vi "Velociprobe_Nanopositioner_Control_RT 3.vi"() -> ()   [LabVIEW 2015] (continued)
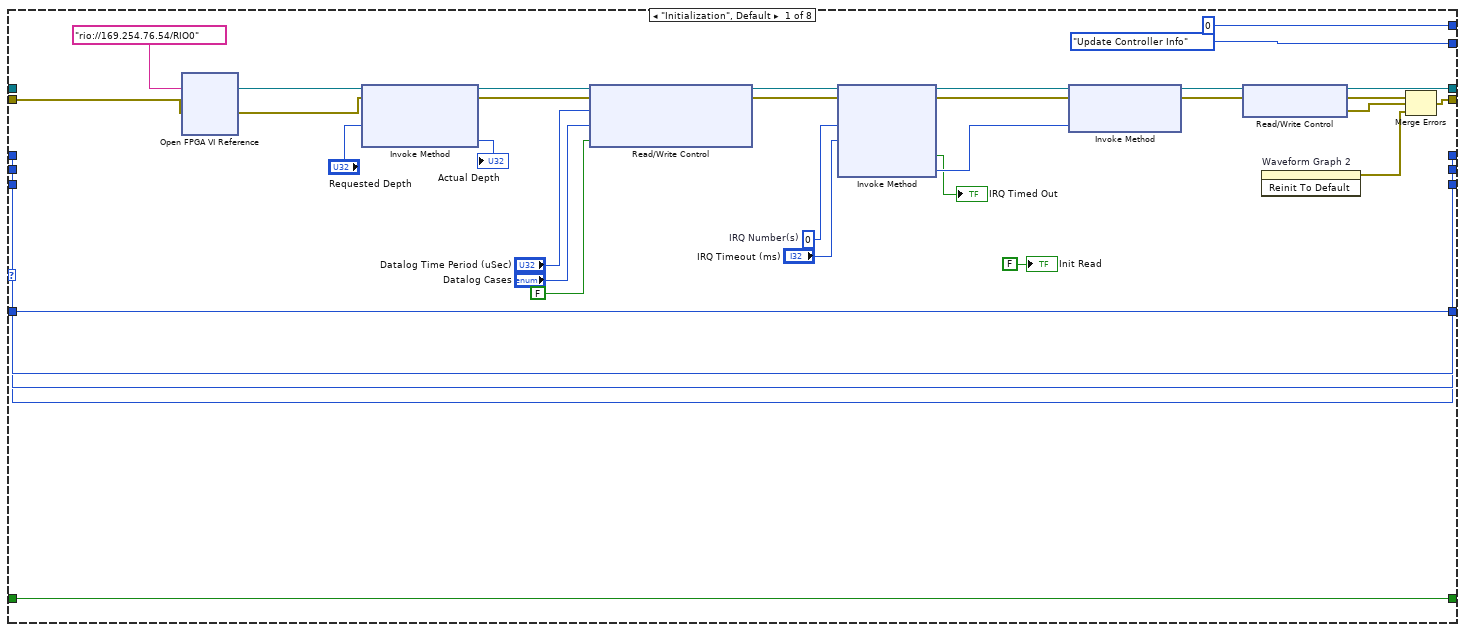
[diagram p2: hidden frame]
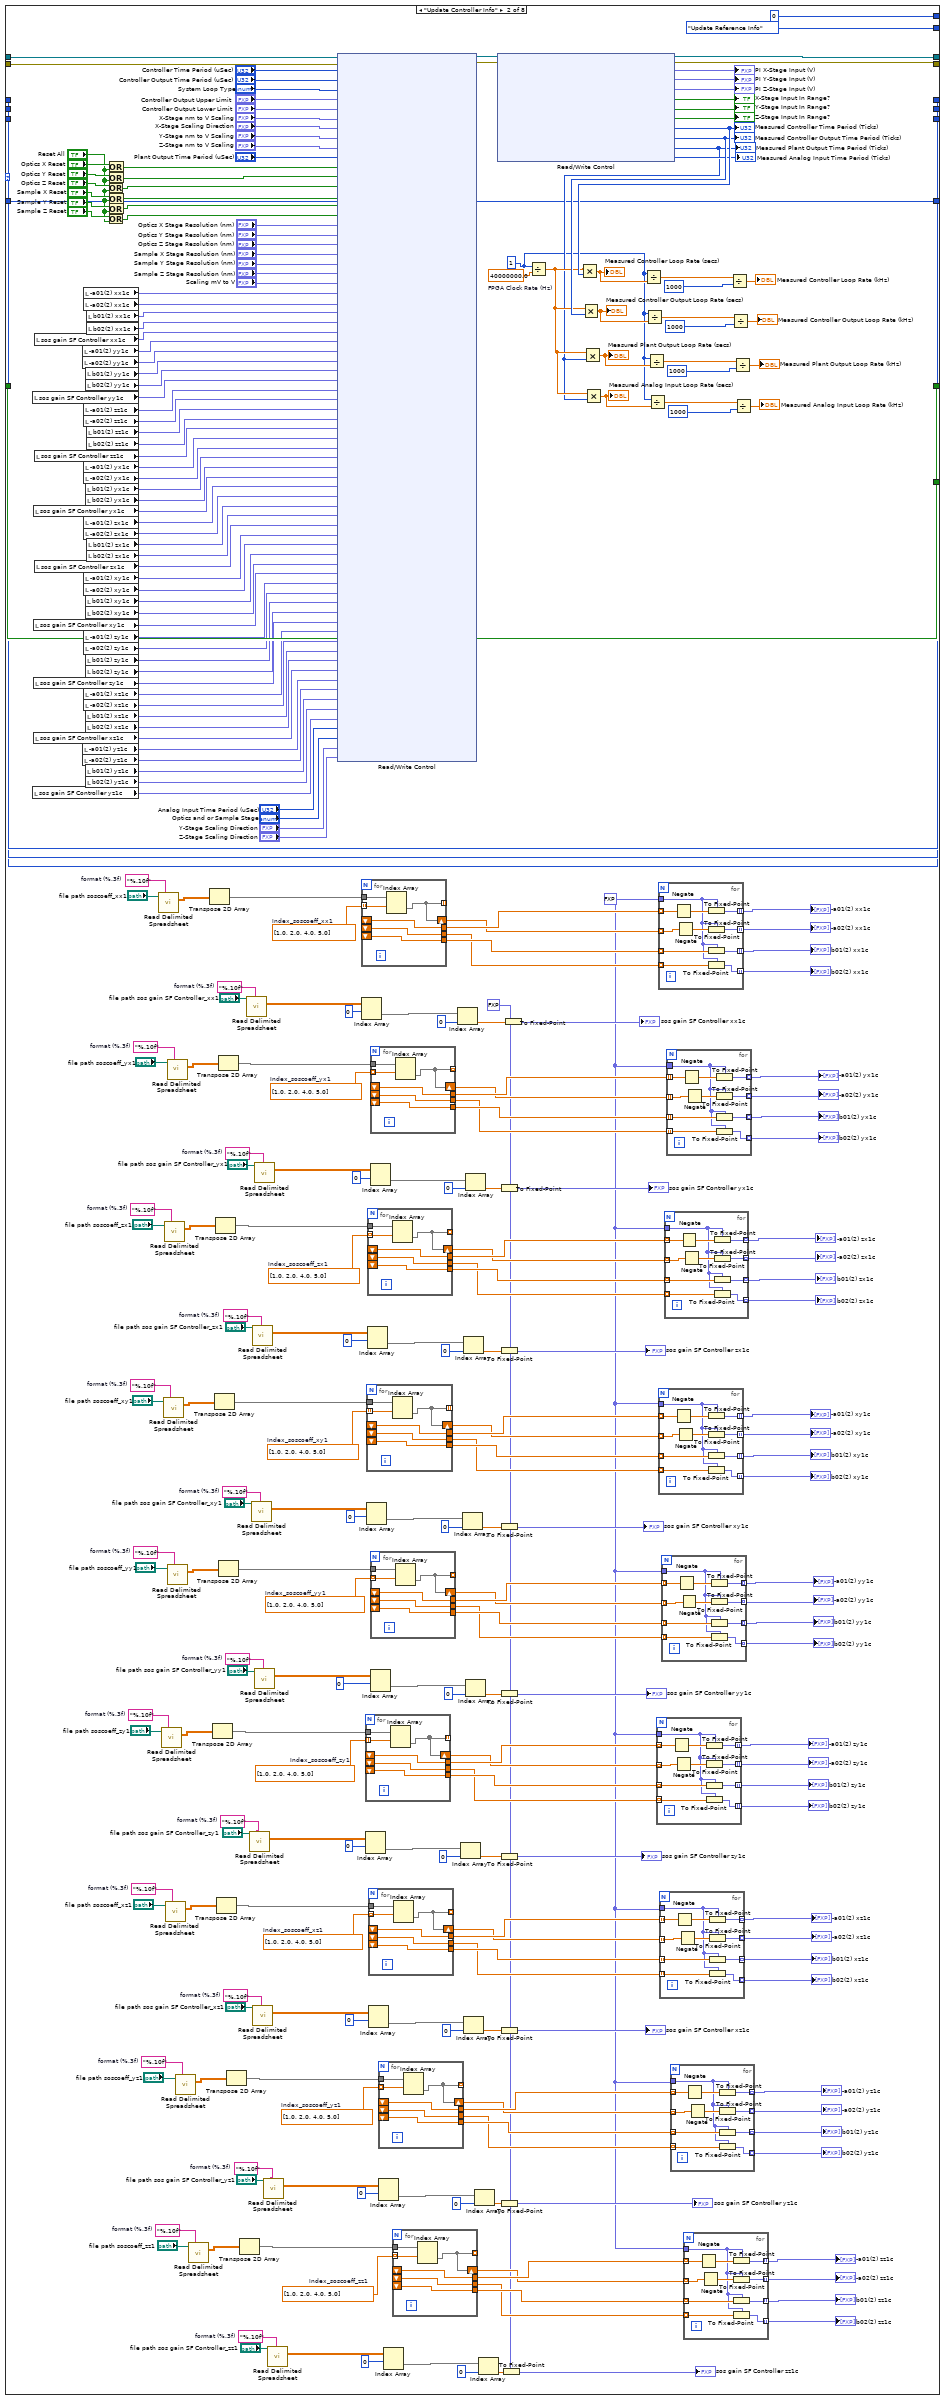
[diagram p3: hidden frame]
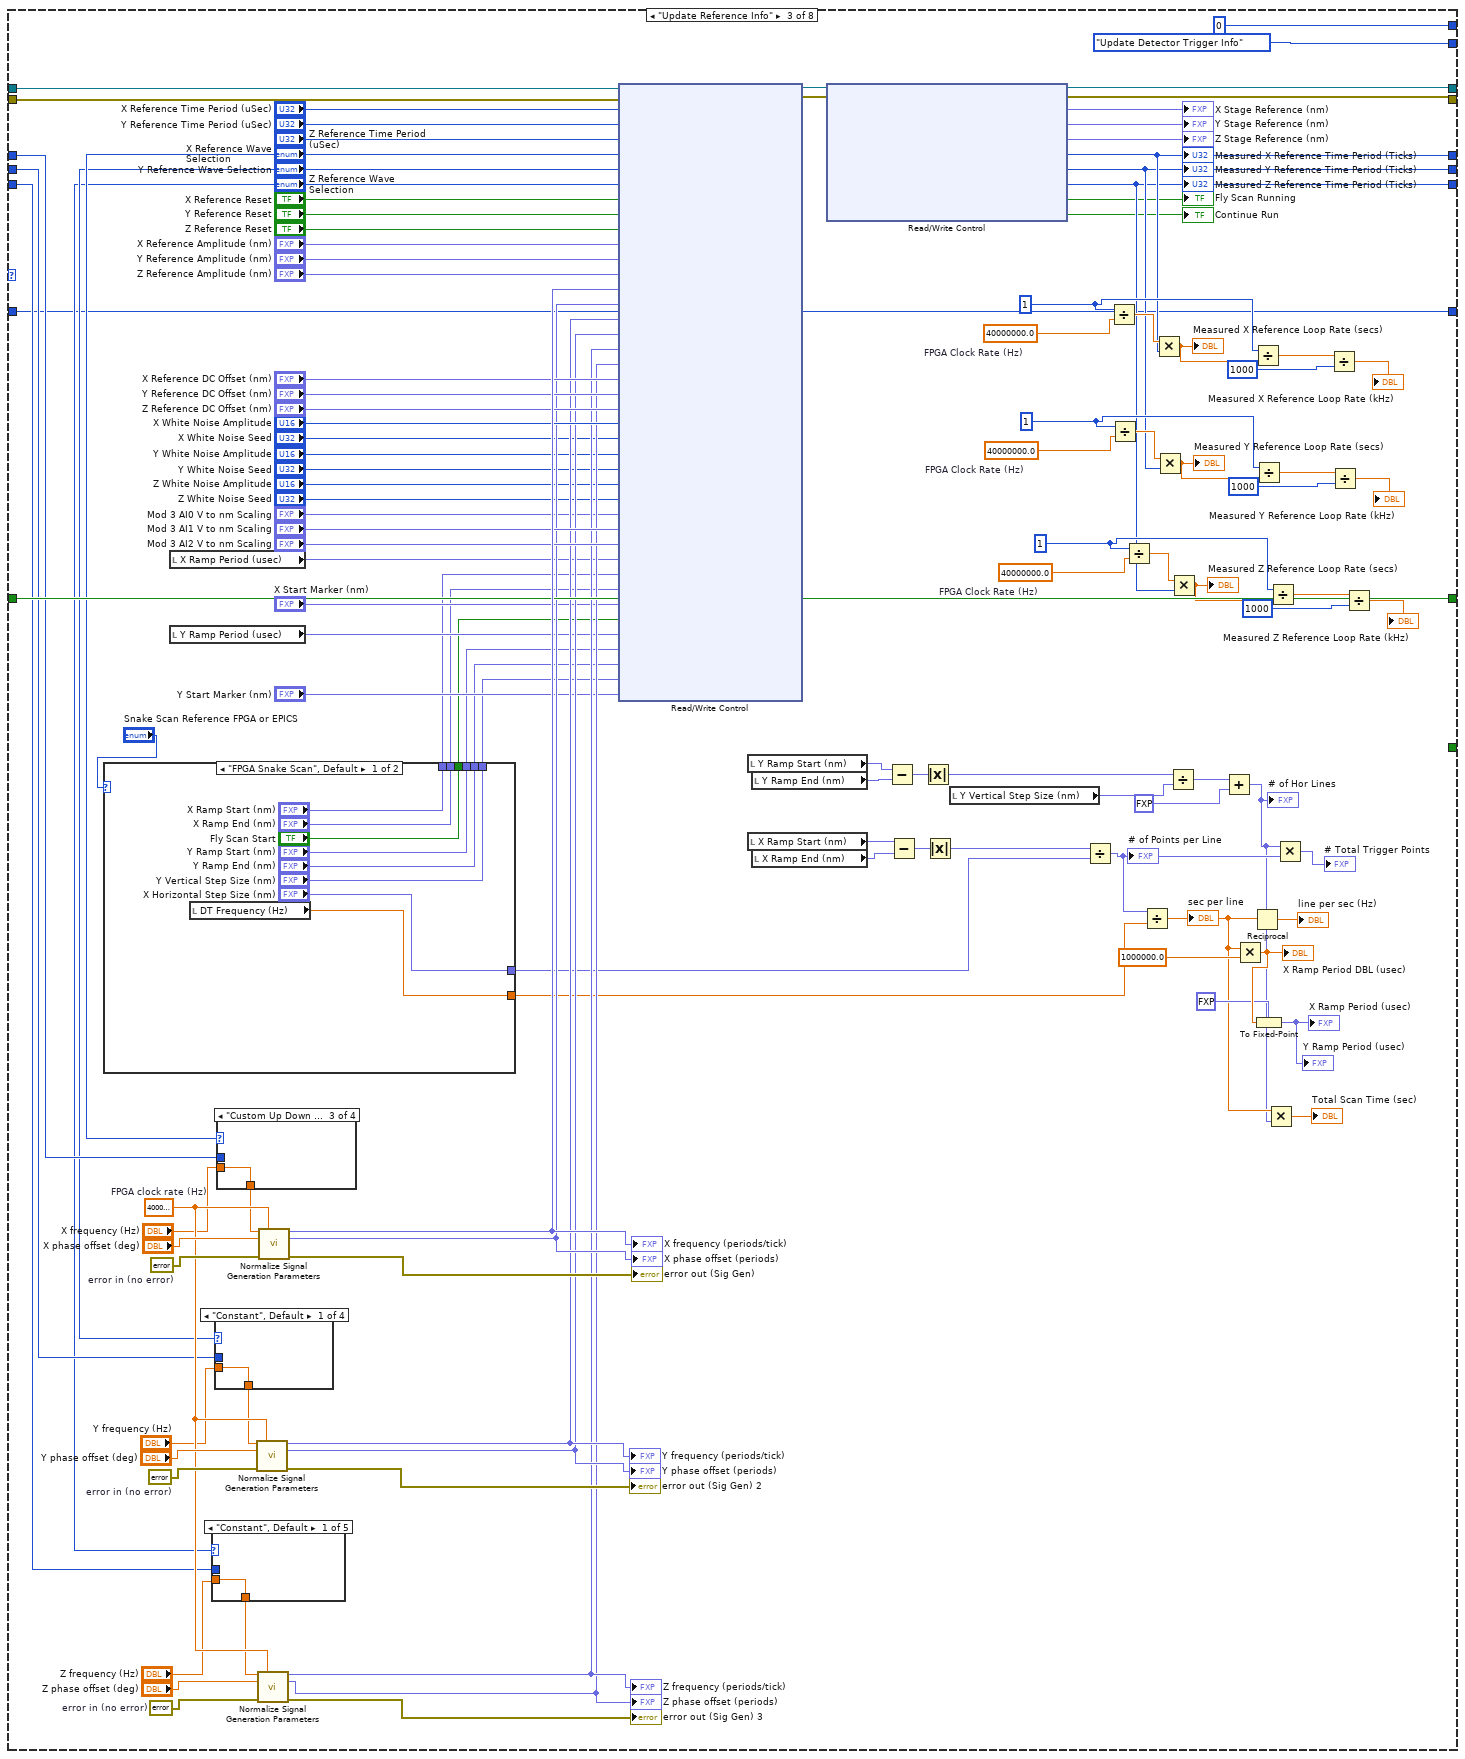
[diagram p4: hidden frame]
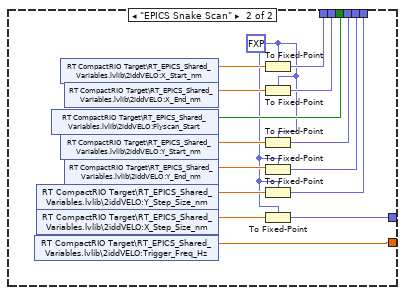
[diagram p5: hidden frame]
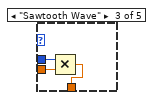
[diagram p7: hidden frame]
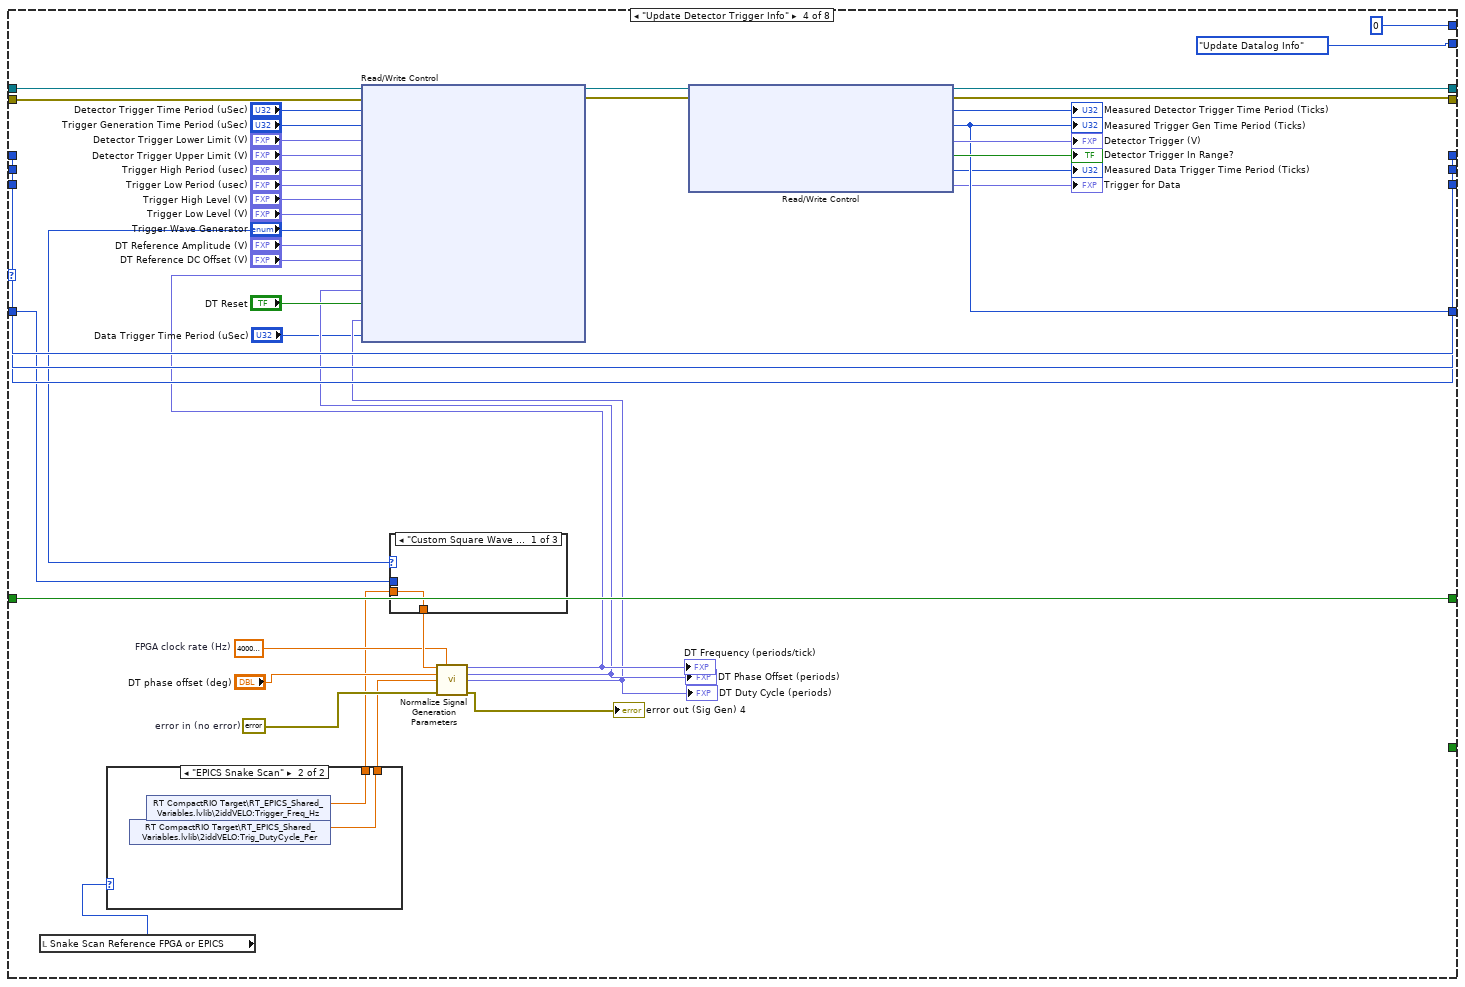
[diagram p16: hidden frame]
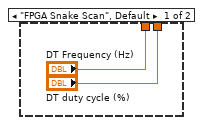
[diagram p17: hidden frame]
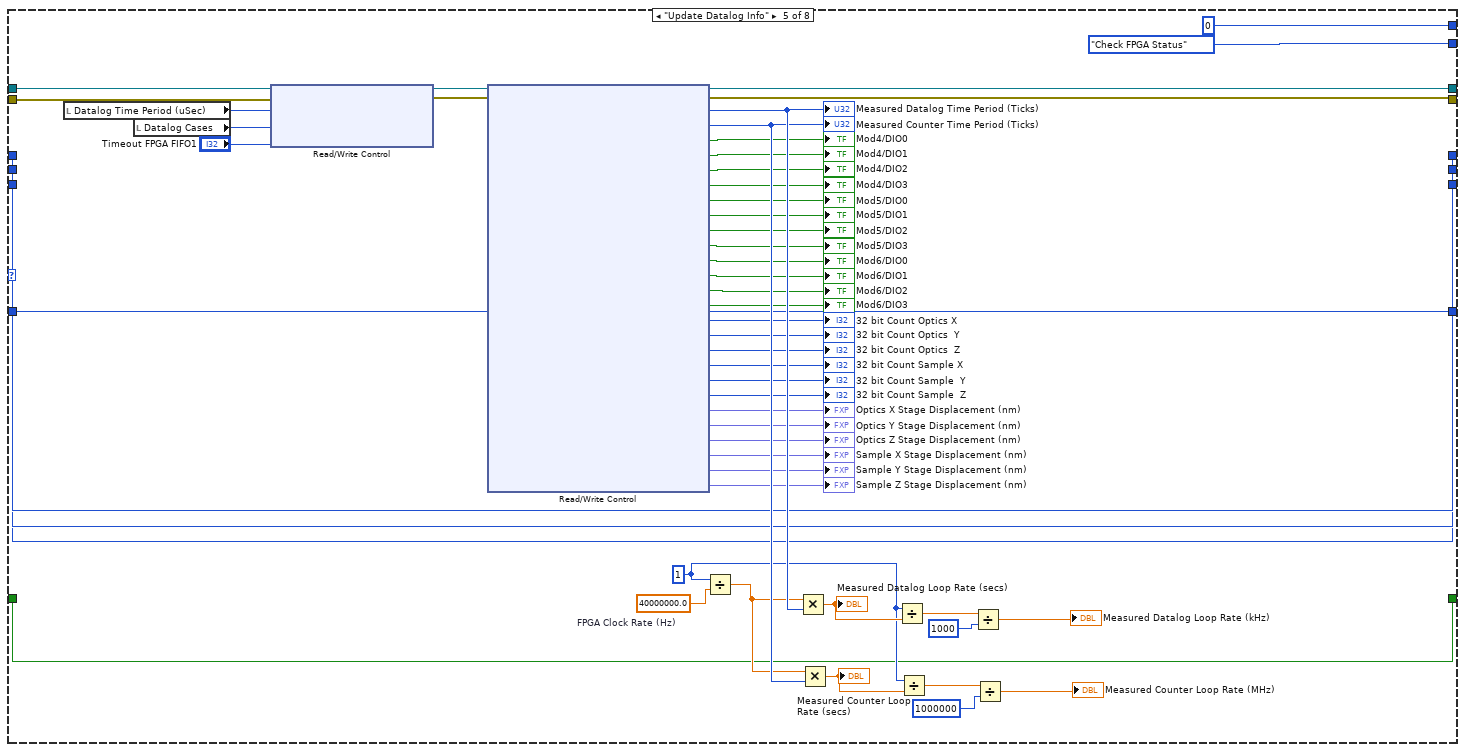
[diagram p20: hidden frame]
            n221 = shared-variable "RT CompactRIO Target\\RT_EPICS_Shared_Variables.lvlib\\2iddVELO:Flyscan_Start"() -> (w667:bool)  [unwired: 1 in, 1 out]
            n222 = shared-variable "RT CompactRIO Target\\RT_EPICS_Shared_Variables.lvlib\\2iddVELO:X_Start_nm"() -> (w675:dbl)  [unwired: 1 in, 1 out]
            n223 = shared-variable "RT CompactRIO Target\\RT_EPICS_Shared_Variables.lvlib\\2iddVELO:Y_Start_nm"() -> (w673:dbl)  [unwired: 1 in, 1 out]
            n224 = shared-variable "RT CompactRIO Target\\RT_EPICS_Shared_Variables.lvlib\\2iddVELO:X_End_nm"() -> (w674:dbl)  [unwired: 1 in, 1 out]
            n225 = shared-variable "RT CompactRIO Target\\RT_EPICS_Shared_Variables.lvlib\\2iddVELO:Y_End_nm"() -> (w672:dbl)  [unwired: 1 in, 1 out]
            n226 = To Fixed-Point(fixed-point type=w662, number=w675) -> (fixed-point=w669:fxp<+/-,16,16>)
            n227 = To Fixed-Point(fixed-point type=w662, number=w674) -> (fixed-point=w668:fxp<+/-,16,16>)
            n228 = To Fixed-Point(fixed-point type=w662, number=w673) -> (fixed-point=w666:fxp<+/-,16,16>)
            n229 = To Fixed-Point(fixed-point type=w662, number=w672) -> (fixed-point=w665:fxp<+/-,16,16>)
            n230 = To Fixed-Point(fixed-point type=w662, number=w671) -> (fixed-point=w664:fxp<+/-,16,16>)
            n231 = To Fixed-Point(fixed-point type=w662, number=w670) -> (fixed-point=w663:fxp<+/-,16,16>)
          }
        }
        n232 = local read "X Ramp Period (usec)"() -> (w551:fxp<+,24,24>)
        n233 = local read "Y Ramp Period (usec)"() -> (w552:fxp<+,24,24>)
        n234 = case shown="\"Constant\", Default" "Z Reference Wave Selection" {
          tunnel: "Z frequency (Hz)" -> [w676 w677 w679 w681 w682]
          tunnel: [w676 w677 w678 w681 w682] -> w577
          tunnel: w576 -> [_ _ w680 _ _]
          frame "Constant", Default {
          }
          frame "Sine Wave" {
          }
          frame "Sawtooth Wave" {
            n235 = Multiply(x=w680, y=w679) -> (x*y=w678:dbl)
          }
          frame "Square Wave" {
          }
          frame "Filtered White Noise" {
          }
        }
        n236 = case shown="\"Constant\", Default" "Y Reference Wave Selection" {
          tunnel: "Y frequency (Hz)" -> [w683 w684 w685 w686]
          tunnel: [w683 w684 w685 w686] -> w582
          tunnel: w579 -> [_ _ _ _]
          frame "Constant", Default {
          }
          frame "Sine Wave" {
          }
          frame "Custom Ramp Wave" {
          }
          frame "Filtered White Noise" {
          }
        }
        n237 = case shown="\"Custom Up Down Ramp\"" "X Reference Wave Selection" {
          tunnel: "X frequency (Hz)" -> [w687 w688 w689 w690]
          tunnel: [w687 w688 w689 w690] -> w586
          tunnel: w584 -> [_ _ _ _]
          frame "Constant", Default {
          }
          frame "Sine Wave" {
          }
          frame "Custom Up Down Ramp" {
          }
          frame "Filtered White Noise" {
          }
        }
        n238 = call <vilib>:"Normalize Signal Generation Parameters.vi"("frequency (Hz)"=w582, "FPGA clock rate (Hz)"=w616, "phase offset (deg)"="Y phase offset (deg)", "error in (no error)"=w623) -> ("frequency (periods/tick)"=w619:fxp<+,32,0>, "phase offset (periods)"=w618:fxp<+,32,0>, "error out"=→"error out (Sig Gen) 2":errorcluster)  [unwired: 6 in, 3 out]
        "Y frequency (periods/tick)" <- w619
        "Y phase offset (periods)" <- w618
        n239 = call <vilib>:"Normalize Signal Generation Parameters.vi"("frequency (Hz)"=w577, "FPGA clock rate (Hz)"=w616, "phase offset (deg)"="Z phase offset (deg)", "error in (no error)"=w620) -> ("frequency (periods/tick)"=w617:fxp<+,32,0>, "phase offset (periods)"=w595:fxp<+,32,0>, "error out"=→"error out (Sig Gen) 3":errorcluster)  [unwired: 6 in, 3 out]
        "Z frequency (periods/tick)" <- w617
        "Z phase offset (periods)" <- w595
        n240 = call <vilib>:"Normalize Signal Generation Parameters.vi"("frequency (Hz)"=w586, "FPGA clock rate (Hz)"=w616, "phase offset (deg)"="X phase offset (deg)", "error in (no error)"=w649) -> ("frequency (periods/tick)"=w648:fxp<+,32,0>, "phase offset (periods)"=w626:fxp<+,32,0>, "error out"=→"error out (Sig Gen)":errorcluster)  [unwired: 6 in, 3 out]
        "X frequency (periods/tick)" <- w648
        "X phase offset (periods)" <- w626
        n241 = xnode "Read/Write Control"("FPGA VI Reference In"=w536, "error in"=w535, "X Reference Time Period (uSec)"="X Reference Time Period (uSec)", "Y Reference Time Period (uSec)"="Y Reference Time Period (uSec)", "Z Reference Time Period (uSec)"="Z Reference Time Period (uSec)", "X Reference Wave Selection"="X Reference Wave Selection", "Y Reference Wave Selection"="Y Reference Wave Selection", "Z Reference Wave Selection"="Z Reference Wave Selection", "X Reference Reset"="X Reference Reset", "Y Reference Reset"="Y Reference Reset", "Z Reference Reset"="Z Reference Reset", "X Reference Amplitude (nm)"="X Reference Amplitude (nm)", "Y Reference Amplitude (nm)"="Y Reference Amplitude (nm)", "Z Reference Amplitude (nm)"="Z Reference Amplitude (nm)", "X Frequency (periods/tick)"=w648, "X Phase Offset (periods)"=w626, "Y Frequency (periods/tick)"=w619, "Y Phase Offset (periods)"=w618, "Z Frequency (periods/tick)"=w617, "Z Phase Offset (periods)"=w595, "X Reference DC Offset (nm)"="X Reference DC Offset (nm)", "Y Reference DC Offset (nm)"="Y Reference DC Offset (nm)", "Z Reference DC Offset (nm)"="Z Reference DC Offset (nm)", "X White Noise Amplitude"="X White Noise Amplitude", "X White Noise Seed"="X White Noise Seed", "Y White Noise Amplitude"="Y White Noise Amplitude", "Y White Noise Seed"="Y White Noise Seed", "Z White Noise Amplitude"="Z White Noise Amplitude", "Z White Noise Seed"="Z White Noise Seed", "Mod 3 AI0 V to nm Scaling"="Mod 3 AI0 V to nm Scaling", "Mod 3 AI1 V to nm Scaling"="Mod 3 AI1 V to nm Scaling", "Mod 3 AI2 V to nm Scaling"="Mod 3 AI2 V to nm Scaling", "X Ramp Period (usec)"=w551, "X Ramp Start (nm)"=w544, "X Ramp End (nm)"=w543, "X Start Marker (nm)"="X Start Marker (nm)", "Fly Scan Start"=w542, "Y Ramp Period (usec)"=w552, "Y Ramp Start (nm)"=w541, "Y Ramp End (nm)"=w540, "Y Ramp Drop Size (nm)"=w539, "Y Start Marker (nm)"="Y Start Marker (nm)") -> ("FPGA VI Reference Out"=w534:refnum<k20>, "error out"=w533:errorcluster)
        n242 = local read "Y Ramp Start (nm)"() -> (w550:fxp<+/-,16,16>)
        n243 = local read "X Ramp Start (nm)"() -> (w548:fxp<+/-,16,16>)
        n244 = local read "Y Ramp End (nm)"() -> (w549:fxp<+/-,16,16>)
        n245 = local read "X Ramp End (nm)"() -> (w547:fxp<+/-,16,16>)
        n246 = xnode "Read/Write Control"("FPGA VI Reference In"=w534, "error in"=w533) -> ("FPGA VI Reference Out"=w531:refnum<k20>, "error out"=w532:errorcluster, "X Stage Reference (nm)"=→"X Stage Reference (nm)":fxp<+/-,58,25>, "Y Stage Reference (nm)"=→"Y Stage Reference (nm)":fxp<+/-,58,25>, "Z Stage Reference (nm)"=→"Z Stage Reference (nm)":fxp<+/-,58,25>, "Measured X Reference Time Period (Ticks)"=w585:u32, "Measured Y Reference Time Period (Ticks)"=w581:u32, "Measured Z Reference Time Period (Ticks)"=w580:u32, "Fly Scan Running"=→"Fly Scan Running":bool, "Continue Run"=→"Continue Run":bool)
        "Measured X Reference Time Period (Ticks)" <- w585
        "Measured Y Reference Time Period (Ticks)" <- w581
        "Measured Z Reference Time Period (Ticks)" <- w580
        n247 = Subtract(x=w550, y=w549) -> (x-y=w568:fxp<+/-,17,17>)
        n248 = Subtract(x=w548, y=w547) -> (x-y=w566:fxp<+/-,17,17>)
        n249 = Absolute Value(x=w568) -> (abs(x)=w559:fxp<+,16,16>)
        n250 = Absolute Value(x=w566) -> (abs(x)=w565:fxp<+,16,16>)
        n251 = local read "Y Vertical Step Size (nm)"() -> (w546:fxp<+/-,16,16>)
        n252 = Divide(x=w565, y=w538) -> (x/y=w563:fxp<+/-,33,17>)
        "# of Points per Line" <- w563
        n253 = Divide(x=w631, y=w637) -> (x/y=w632:dbl)
        n254 = Divide(x=w609, y=w615) -> (x/y=w610:dbl)
        n255 = Divide(x=w602, y=w608) -> (x/y=w603:dbl)
        n256 = Divide(x=w563, y=w537) -> (x/y=w555:dbl)
        "sec per line" <- w555
        n257 = Multiply(x=w632, y=w585) -> (x*y=w636:dbl)
        "Measured X Reference Loop Rate (secs)" <- w636
        n258 = Multiply(x=w610, y=w581) -> (x*y=w614:dbl)
        "Measured Y Reference Loop Rate (secs)" <- w614
        n259 = Divide(x=w559, y=w546) -> (x/y=w560:fxp<+/-,33,17>)
        n260 = Multiply(x=w603, y=w580) -> (x*y=w607:dbl)
        "Measured Z Reference Loop Rate (secs)" <- w607
        n261 = Add(x=w560, y=fxp<+,16,16> 1.0) -> (x+y=w554:fxp<+/-,34,18>)
        "# of Hor Lines" <- w554
        n262 = Multiply(x=w555, y=1000000.0) -> (x*y=w558:dbl)
        "X Ramp Period DBL (usec)" <- w558
        n263 = Reciprocal(x=w555) -> (1/x=→"line per sec (Hz)":dbl)
        n264 = Divide(x=w631, y=w636) -> (x/y=w635:dbl)
        n265 = Divide(x=w609, y=w614) -> (x/y=w613:dbl)
        n266 = To Fixed-Point(fixed-point type=fxp<+,24,24> 0.0, number=w558) -> (fixed-point=→"X Ramp Period (usec)" →"Y Ramp Period (usec)":fxp<+,24,24>)
        n267 = Multiply(x=w555, y=w554) -> (x*y=→"Total Scan Time (sec)":dbl)
        n268 = Divide(x=w602, y=w607) -> (x/y=w606:dbl)
        n269 = Multiply(x=w554, y=w563) -> (x*y=→"# Total Trigger Points":fxp<+/-,64,34>)
        n270 = Divide(x=w635, y=1000) -> (x/y=→"Measured X Reference Loop Rate (kHz)":dbl)
        n271 = Divide(x=w613, y=1000) -> (x/y=→"Measured Y Reference Loop Rate (kHz)":dbl)
        n272 = Divide(x=w606, y=1000) -> (x/y=→"Measured Z Reference Loop Rate (kHz)":dbl)
      }
      frame "Update Detector Trigger Info" {
        w709 = 40000000.0  # FPGA clock rate (Hz)
        w711 = errorcluster {"status"=FALSE, "code"=0, "source"=""}  # error in (no error)
        n273 = local read "Snake Scan Reference FPGA or EPICS"() -> (w702:enum16{"FPGA Snake Scan", "EPICS Snake Scan"})
        n274 = case shown="\"EPICS Snake Scan\"" w702 {
          tunnel: ["DT Frequency (Hz)" w737] -> w701
          tunnel: ["DT duty cycle (%)" w736] -> w700
          frame "FPGA Snake Scan", Default {
          }
          frame "EPICS Snake Scan" {
            n275 = shared-variable "RT CompactRIO Target\\RT_EPICS_Shared_Variables.lvlib\\2iddVELO:Trig_DutyCycle_Per"() -> (w736:dbl)  [unwired: 1 in, 1 out]
            n276 = shared-variable "RT CompactRIO Target\\RT_EPICS_Shared_Variables.lvlib\\2iddVELO:Trigger_Freq_Hz"() -> (w737:dbl)  [unwired: 1 in, 1 out]
          }
        }
        n277 = case shown="\"Custom Square Wave \", Default" "Trigger Wave Generator" {
          tunnel: w701 -> [w738 w739 w740]
          tunnel: [w738 w739 w740] -> w710
          tunnel: w703 -> [_ _ _]
          frame "Custom Square Wave ", Default {
          }
          frame "Square Wave 1" {
          }
          frame "Square Wave 2" {
          }
        }
        n278 = call <vilib>:"Normalize Signal Generation Parameters.vi"("frequency (Hz)"=w710, "FPGA clock rate (Hz)"=w709, "phase offset (deg)"="DT phase offset (deg)", "duty cycle (%)"=w700, "error in (no error)"=w711) -> ("frequency (periods/tick)"=w707:fxp<+,32,0>, "phase offset (periods)"=w706:fxp<+,32,0>, "duty cycle (periods)"=w705:fxp<+,32,0>, "error out"=→"error out (Sig Gen) 4":errorcluster)  [unwired: 5 in, 2 out]
        "DT Frequency (periods/tick)" <- w707
        "DT Phase Offset (periods)" <- w706
        "DT Duty Cycle (periods)" <- w705
        n279 = xnode "Read/Write Control"("FPGA VI Reference In"=w699, "error in"=w698, "Detector Trigger Time Period (uSec)"="Detector Trigger Time Period (uSec)", "Trigger Generation Time Period (uSec)"="Trigger Generation Time Period (uSec)", "Detector Trigger Lower Limit (V)"="Detector Trigger Lower Limit (V)", "Detector Trigger Upper Limit (V)"="Detector Trigger Upper Limit (V)", "Trigger High Period (usec)"="Trigger High Period (usec)", "Trigger Low Period (usec)"="Trigger Low Period (usec)", "Trigger High Level (V)"="Trigger High Level (V)", "Trigger Low Level (V)"="Trigger Low Level (V)", "Trigger Wave Generator"="Trigger Wave Generator", "DT Reference Amplitude (V)"="DT Reference Amplitude (V)", "DT Reference DC Offset (V)"="DT Reference DC Offset (V)", "DT Frequency (periods/tick)"=w707, "DT Phase Offset (periods)"=w706, "DT Reset"="DT Reset", "DT Duty Cycle (periods)"=w705, "Data Trigger Time Period (uSec)"="Data Trigger Time Period (uSec)") -> ("FPGA VI Reference Out"=w697:refnum<k20>, "error out"=w696:errorcluster)
        n280 = xnode "Read/Write Control"("FPGA VI Reference In"=w697, "error in"=w696) -> ("FPGA VI Reference Out"=w695:refnum<k20>, "error out"=w694:errorcluster, "Measured Detector Trigger Time Period (Ticks)"=→"Measured Detector Trigger Time Period (Ticks)":u32, "Measured Trigger Gen Time Period (Ticks)"=w704:u32, "Detector Trigger (V)"=→"Detector Trigger (V)":fxp<+/-,20,5>, "Detector Trigger In Range?"=→"Detector Trigger In Range?":bool, "Measured Data Trigger Time Period (Ticks)"=→"Measured Data Trigger Time Period (Ticks)":u32, "Trigger for Data"=→"Trigger for Data":fxp<+/-,58,25>)
        "Measured Trigger Gen Time Period (Ticks)" <- w704
      }
      frame "Update Datalog Info" {
        w785 = 40000000.0  # FPGA Clock Rate (Hz)
        w774 = 1
        n281 = local read "Datalog Time Period (uSec)"() -> (w772:u32)
        n282 = local read "Datalog Cases"() -> (w771:T6)
        n283 = xnode "Read/Write Control"("FPGA VI Reference In"=w746, "error in"=w745, "Datalog Time Period (uSec)"=w772, "Datalog Cases"=w771, "Timeout FPGA FIFO1"="Timeout FPGA FIFO1") -> ("FPGA VI Reference Out"=w744:refnum<k20>, "error out"=w743:errorcluster)
        n284 = xnode "Read/Write Control"("FPGA VI Reference In"=w744, "error in"=w743) -> ("FPGA VI Reference Out"=w741:refnum<k20>, "error out"=w742:errorcluster, "Measured Datalog Time Period (Ticks)"=w784:u32, "Measured Counter Time Period (Ticks)"=w782:u32, "Mod4/DIO0"=→"Mod4/DIO0":bool, "Mod4/DIO1"=→"Mod4/DIO1":bool, "Mod4/DIO2"=→"Mod4/DIO2":bool, "Mod4/DIO3"=→"Mod4/DIO3":bool, "Mod5/DIO0"=→"Mod5/DIO0":bool, "Mod5/DIO1"=→"Mod5/DIO1":bool, "Mod5/DIO2"=→"Mod5/DIO2":bool, "Mod5/DIO3"=→"Mod5/DIO3":bool, "Mod6/DIO0"=→"Mod6/DIO0":bool, "Mod6/DIO1"=→"Mod6/DIO1":bool, "Mod6/DIO2"=→"Mod6/DIO2":bool, "Mod6/DIO3"=→"Mod6/DIO3":bool, "32 bit Count Optics X"=→"32 bit Count Optics X":i32, "32 bit Count Optics  Y"=→"32 bit Count Optics  Y":i32, "32 bit Count Optics  Z"=→"32 bit Count Optics  Z":i32, "32 bit Count Sample X"=→"32 bit Count Sample X":i32, "32 bit Count Sample  Y"=→"32 bit Count Sample  Y":i32, "32 bit Count Sample  Z"=→"32 bit Count Sample  Z":i32, "Optics X Stage Displacement (nm)"=→"Optics X Stage Displacement (nm)":fxp<+/-,58,25>, "Optics Y Stage Displacement (nm)"=→"Optics Y Stage Displacement (nm)":fxp<+/-,58,25>, "Optics Z Stage Displacement (nm)"=→"Optics Z Stage Displacement (nm)":fxp<+/-,58,25>, "Sample X Stage Displacement (nm)"=→"Sample X Stage Displacement (nm)":fxp<+/-,58,25>, "Sample Y Stage Displacement (nm)"=→"Sample Y Stage Displacement (nm)":fxp<+/-,58,25>, "Sample Z Stage Displacement (nm)"=→"Sample Z Stage Displacement (nm)":fxp<+/-,58,25>)
        "Measured Datalog Time Period (Ticks)" <- w784
        "Measured Counter Time Period (Ticks)" <- w782
        n285 = Divide(x=w774, y=w785) -> (x/y=w781:dbl)
        n286 = Multiply(x=w781, y=w784) -> (x*y=w792:dbl)
        "Measured Datalog Loop Rate (secs)" <- w792
        n287 = Multiply(x=w781, y=w782) -> (x*y=w788:dbl)
        "Measured Counter Loop Rate (secs)" <- w788
        n288 = Divide(x=w774, y=w792) -> (x/y=w791:dbl)
        n289 = Divide(x=w774, y=w788) -> (x/y=w787:dbl)
        n290 = Divide(x=w791, y=1000) -> (x/y=→"Measured Datalog Loop Rate (kHz)":dbl)
        n291 = Divide(x=w787, y=1000000) -> (x/y=→"Measured Counter Loop Rate (MHz)":dbl)
      }
      frame "Check FPGA Status" {
        n292 = xnode "Read/Write Control"("FPGA VI Reference In"=w798, "error in"=w797) -> ("FPGA VI Reference Out"=w796:refnum<k20>, "error out"=w795:errorcluster, "error out (FPGA)"=w811:errorcluster, "error out (AO FPGA)"=w810:errorcluster, "FIFO Timed Out?"=→"FIFO Timed Out?":bool, "stop case"=w805:bool, "FIFO Timed Out"=w804:bool)
        "error out (FPGA)" <- w811
        "error out (AO FPGA)" <- w810
        "stop case" <- w805
        "FIFO Timed Out" <- w804
        n293 = Merge Errors "Merge Errors"(w795, w811, w810) -> (w806:errorcluster)
        n294 = Unbundle By Name "Unbundle By Name"(w806) -> ("status"=w809:bool)
        n295 = Compound Arithmetic op=OR(w809, w805, w804) -> (w807:bool)
        n296 = Bundle By Name "Bundle By Name"(cluster=w806, "status"=w807) -> (w794:errorcluster)
      }
      frame "Reading FIFO" {
        w814 = ","  # delimiter (Tab)
        w818 = 0.0  # t0
        w819 = "%8f"  # format string
        w873 = 0.0  # t0
        n297 = local read "Snake Scan Reference FPGA or EPICS"() -> (w824:enum16{"FPGA Snake Scan", "EPICS Snake Scan"})
        n298 = xnode "Read/Write Control"("FPGA VI Reference In"=w831, "error in"=w823) -> ("FPGA VI Reference Out"=w830:refnum<k20>, "error out"=w829:errorcluster, "Number of Data Strings"=→"Number of Data Strings":i32)
        n299 = case shown="\"FPGA Snake Scan\", Default" w824 {
          tunnel: ["Write Data" w885] -> w860
          frame "FPGA Snake Scan", Default {
          }
          frame "EPICS Snake Scan" {
            n300 = shared-variable "RT CompactRIO Target\\RT_EPICS_Shared_Variables.lvlib\\2iddVELO:Write_Data"() -> (w885:bool)  [unwired: 1 in, 1 out]
          }
        }
        n301 = local read "Init Read"() -> (w821:bool)
        n302 = case shown="True" w821 {
          tunnel: w823 -> [_ w882]
          tunnel: [_ w881] -> w822
          tunnel: [_ w879] -> w820
          frame False {
          }
          frame True {
            n303 = call "Data_Read.vi"("file (use dialog)"="file (use dialog)", "Data Read Count"="Data Read Count", "Data Read Control"=Data_Read_Control."Read", "error initialize"=w882) -> ("Read text"=w879:string, "Read Cancelled"=→"Read Cancelled":bool, "error out"=w881:errorcluster)  [unwired: 3 in]
            "Read text" <- w879
          }
        }
        n304 = Greater?(x=w860, y=w859) -> (0:w856:bool)
        n305 = case shown="True" w856 {
          tunnel: w823 -> [w900 w904]
          tunnel: [w900 w905] -> w854
          frame False {
          }
          frame True {
            n306 = local write "Init Read"(FALSE ("Init Read")) -> ()
            n307 = call "Data_Write_2.vi"("Command List"=Data_Write_Control."Initialize", "name"="name", "error initialize"=w904) -> ("error out"=w905:errorcluster)  [unwired: 5 in, 1 out]
          }
        }
        n308 = local read "Datalog Time Period (uSec)"() -> (w871:u32)
        n309 = Less?(x=w860, y=w859) -> (x < y?=w855:bool)
        n310 = Spreadsheet String To Array(delimiter (Tab)=w814, format string=w819, spreadsheet string=w820) -> (array=w816:dbl[][])  [unwired: 1 in]
        "array" <- w816
        n311 = Multiply(x=1e-06, y=w871) -> (x*y=w815:dbl)
        "Datalog Time Period (sec)" <- w815
        n312 = Divide(x=1.0, y=w815) -> (x/y=w867:dbl)
        "Datalog Rate (Hz)" <- w867
        n313 = Multiply(x="FIFO Time Period", y=w867) -> (x*y=w865:dbl)
        n314 = Multiply(x=5 ("Number of Data Strings 2"), y=w865) -> (x*y=w864:dbl)
        n315 = To Unsigned Long Integer(number=w864) -> (unsigned 32bit integer=w861:u32)
        "Number of Elements" <- w861
        n316 = xnode "Invoke Method"("FPGA VI Reference In"=w830, "error in"=w829, "Number of Elements"=w861, "Timeout (ms)"="Timeout (ms)") -> ("FPGA VI Reference Out"=w828:refnum<k20>, "error out"=w827:errorcluster, "Data"=w862:fxp<+/-,58,25>[], "Elements Remaining"=→"Elements Remaining" →"Elements Remaining Waveform Chart" →"Elements Remaining Waveform Chart 3":u32)
        "Data" <- w862
        n317 = Decimate 1D Array "Decimate 1D Array"(w862) -> (w845:fxp<+/-,58,25>[], w836:fxp<+/-,58,25>[], w835:fxp<+/-,58,25>[], w834:fxp<+/-,58,25>[], w832:fxp<+/-,58,25>[])
        n318 = Build Array "Build Array"(w845, w836, w835, w834, w832) -> (w874:fxp<+/-,58,25>[][])
        n319 = To Double Precision Float(number=w874) -> (double precision float=w869:dbl[][])
        n320 = call "Convert to Dynamic Data"("Array"=w845) -> ("Dynamic Data Type"=w843:dynamicdata)  [unwired: 3 in]
        n321 = call "Convert to Dynamic Data2"("Array"=w836) -> ("Dynamic Data Type"=w837:dynamicdata)  [unwired: 3 in]
        n322 = call "Convert to Dynamic Data3"("Array"=w835) -> ("Dynamic Data Type"=w839:dynamicdata)  [unwired: 3 in]
        n323 = call "Convert to Dynamic Data4"("Array"=w834) -> ("Dynamic Data Type"=w838:dynamicdata)  [unwired: 3 in]
        n324 = Transpose 2D Array(2D array=w869) -> (transposed array=w852:dbl[][])
        n325 = case shown="True" w860 {
          tunnel: w854 -> [w891 w896]
          tunnel: [w891 w895] -> w853
          tunnel: w852 -> [_ w897]
          frame False {
          }
          frame True {
            w899 = "%8f"  # format string
            w898 = ","  # delimiter (Tab)
            n326 = Array To Spreadsheet String(delimiter (Tab)=w898, array=w897, 3:w899) -> (spreadsheet string=w893:string)
            "spreadsheet string" <- w893
            n327 = call "Data_Write_2.vi"("Command List"=Data_Write_Control."Write", "Data"=w893, "error initialize"=w896) -> ("Refnum Out During Write"=→"Refnum Out During Write":refnum<file>, "error out"=w895:errorcluster)  [unwired: 5 in]
          }
        }
        n328 = call "Convert from Dynamic Data"("Dynamic Data Type"=w843) -> ("Array"=w844:dbl[])  [unwired: 3 in]
        n329 = call "Convert from Dynamic Data2"("Dynamic Data Type"=w837) -> ("Array"=w842:dbl[])  [unwired: 3 in]
        n330 = call "Convert from Dynamic Data3"("Dynamic Data Type"=w839) -> ("Array"=w841:dbl[])  [unwired: 3 in]
        n331 = call "Convert from Dynamic Data4"("Dynamic Data Type"=w838) -> ("Array"=w840:dbl[])  [unwired: 3 in]
        n332 = Bundle("Array"=w844, "Array"=w842) -> (→"XY Graph":cluster{"Array":dbl[], "Array":dbl[]})  [unwired: 1 in]
        n333 = Bundle("Array"=w841, "Array"=w840) -> (→"XY Graph 2":cluster{"Array":dbl[], "Array":dbl[]})  [unwired: 1 in]
        n334 = case shown="True" w855 {
          tunnel: w853 -> [w886 w889]
          tunnel: [w886 w888] -> w863
          frame False {
          }
          frame True {
            n335 = local write "Init Read"(TRUE ("Init Read")) -> ()
            n336 = call "Data_Write_2.vi"("Command List"=Data_Write_Control."Close", "error initialize"=w889) -> ("error out"=w888:errorcluster)  [unwired: 6 in, 1 out]
          }
        }
        n337 = Bundle("t0"=w873, w815, w869) -> (→"Waveform Graph 2":cluster{"t0":dbl, dbl, dbl[][]})  [unwired: 1 in]
        n338 = Bundle("t0"=w818, w815, w816) -> (→"Waveform Graph 3":cluster{"t0":dbl, dbl, dbl[][]})  [unwired: 1 in]
        n339 = Merge Errors "Merge Errors"(w827, w863, w822) -> (w826:errorcluster)
      }
      frame "Exit" {
        w918 = TRUE ("Stop")
        n340 = xnode "Invoke Method"("FPGA VI Reference In"=w912, "error in"=w911) -> ("FPGA VI Reference Out"=w910:refnum<k20>, "error out"=w909:errorcluster)
        n341 = xnode "Read/Write Control"("FPGA VI Reference In"=w910, "error in"=w909, "stop case"=TRUE) -> ("FPGA VI Reference Out"=w908:refnum<k20>, "error out"=w907:errorcluster)
        n342 = local write "Stop"(w918) -> ()
        n343 = xnode "Close FPGA VI Reference"("FPGA VI Reference In"=w908, "error in"=w907) -> ("error out"=w906:errorcluster)
      }
    }
    n344 = call "State Control.vi"("Error Input"=w14, "Input States"=w25, "Stop"="Stop") -> ("Output State"=w24:T7)  [unwired: 8 in]
    n345 = node-c288(w31) -> ()  [unwired: 1 out]
  }
  n346 = node-c288(w7) -> (→"Error (RT)":errorcluster, →"Iteration Duration RT Timed-Loop":i64)
  n347 = call <vilib>:"Simple Error Handler.vi"("error in (no error)"=w1) -> ("message"=→"message":string)  [unwired: 4 in, 4 out]
